vi "UHR-Fleezers Control (host) - 10.7.vi"() -> ()   [LabVIEW 2010] (continued)
          }
        }
        "Raster Scanning..." <- TRUE ("Scanning...")
      }
    }
    n290 = And(x="Save scans", y=w1174) -> (x .and. y?=w1220:bool)
    n291 = Compound Arithmetic op=OR("Start MCL Scan", "Confocal Image", "Confocal Linescan") -> (w1172:bool)
    n292 = And(x="Save Data (MCL)", y=w1172) -> (x .and. y?=w1219:bool)
    n293 = case "Start MCL raster scan" shown="True" w1172 {
      tunnel: w1222 -> [w2230 w2245]
      tunnel: w1221 -> [w2229 w2244]
      tunnel: [w2230 w2240] -> w979
      tunnel: [w2229 w2239] -> w978
      tunnel: [FALSE w2238] -> w1205
      tunnel: "Start MCL Scan" -> [_ w2233]
      tunnel: "Confocal Image" -> [_ w2232]
      tunnel: "Confocal Linescan" -> [_ _]
      frame False {
      }
      frame True {
        w2238 = TRUE
        n294 = case shown="True" "Restart DMA? (MCL)" {
          tunnel: [w2490 w2492] -> w2243
          tunnel: [w2489 w2491] -> w2242
          tunnel: w2245 -> [w2490 w2495]
          tunnel: w2244 -> [w2489 w2494]
          frame False {
          }
          frame True {
            n295 = call "reset FPGA DMA.vi"("error in"=w2494, "FPGA VI Reference In"=w2495) -> ("error out"=w2491:errorcluster, "FPGA VI Reference Out"=w2492:T19)
            n296 = local write "Overflow (data lost)"(FALSE ("Overflow (data lost)")) -> ()
          }
        }
        n297 = case shown="False" w2233 {
          selector: w2233 -> [_ w2249]
          tunnel: w2232 -> [w2248 _]
          tunnel: [w2248 w2249] -> w2231
          frame False {
            n298 = property on="2D or 1D Scan" class="Bool (strict)"("Val(Sgnl)"=w2248) -> ()  [unwired: 2 in, 2 out]
            n299 = property on="Confocal Image" class="Bool (strict)"("Value"=FALSE ("Start Confocal Map")) -> ()  [unwired: 2 in, 2 out]
          }
          frame True {
          }
        }
        n300 = local write "MCL Scanning"(w2238) -> ()
        n301 = local read "AO1"() -> (w2235:dbl)
        n302 = local read "AO2"() -> (w2234:dbl)
        n303 = case shown="True" "Center Scan" {
          tunnel: w2243 -> [w2256 w2368]
          tunnel: w2242 -> [w2255 w2367]
          tunnel: [w2254 w2366] -> w2240
          tunnel: [w2253 w2365] -> w2239
          tunnel: [w2251 w2352] -> w2237
          tunnel: [w2250 w2351] -> w2236
          tunnel: w2235 -> [w2251 w2357]
          tunnel: w2234 -> [w2250 w2360]
          tunnel: w2231 -> [_ _]
          frame False {
            w2252 = TRUE ("AI to FIFO")
            n304 = xnode "Read/Write Control"("FPGA VI Reference In"=w2256, "error in"=w2255, "AI to FIFO"=w2252, "APD to FIFO"=w2252, "Start scan (MCL)"=w2252) -> ("FPGA VI Reference Out"=w2254:T19, "error out"=w2253:errorcluster)
          }
          frame True {
            w2364 = TRUE ("AI to FIFO")
            n305 = local read "Scan steps (MCL)"() -> (w2343:u64)
            n306 = local read "Scan lines (y)"() -> (w2339:u64)
            n307 = local read "Fast Scan Dir"() -> (w2350:bool)
            n308 = local read "Actual MCL Inc (V)"() -> (w2340:dbl)
            n309 = Decrement(x=w2339) -> (x-1=w2338:u64)
            n310 = Decrement(x=w2343) -> (x-1=w2342:u64)
            n311 = Multiply(x=w2340, y=w2338) -> (x*y=w2337:dbl)
            n312 = Divide(x=w2337, y=2.0) -> (x/y=w2347:dbl)
            n313 = Multiply(x=w2340, y=w2342) -> (x*y=w2341:dbl)
            n314 = Divide(x=w2341, y=2.0) -> (x/y=w2346:dbl)
            n315 = Select(t=w2346, s=w2350, f=w2347) -> (s? t:f=w2345:dbl)
            n316 = Select(t=w2347, s=w2350, f=w2346) -> (s? t:f=w2349:dbl)
            n317 = Subtract(x=w2357, y=w2349) -> (x-y=w2348:dbl)
            n318 = Subtract(x=w2360, y=w2345) -> (x-y=w2344:dbl)
            n319 = local read "2D or 1D Scan"() -> (w2362:bool)
            n320 = Not(x=w2350) -> (.not. x?=w2356:bool)
            n321 = Not(x=w2362) -> (.not. x?=w2358:bool)
            n322 = And(x=w2350, y=w2358) -> (x .and. y?=w2359:bool)
            n323 = And(x=w2358, y=w2356) -> (x .and. y?=w2361:bool)
            n324 = Select(t=w2360, s=w2361, f=w2344) -> (s? t:f=w2351:dbl)
            n325 = Select(t=w2357, s=w2359, f=w2348) -> (s? t:f=w2352:dbl)
            n326 = call "Volt to I16.vi"("Voltage In"=w2352) -> ("I16 Voltage Out"=w2355:i16)
            n327 = call "Volt to I16.vi"("Voltage In"=w2351) -> ("I16 Voltage Out"=w2354:i16)
            n328 = xnode "Read/Write Control"("FPGA VI Reference In"=w2368, "error in"=w2367, "AI to FIFO"=w2364, "APD to FIFO"=w2364, "Start scan (MCL)"=w2364, "AO1"=w2355, "AO2"=w2354) -> ("FPGA VI Reference Out"=w2366:T19, "error out"=w2365:errorcluster)
          }
        }
        "Initial Y" <- w2237
        "Initial X" <- w2236
        "wait to reset values" <- w2238
      }
    }
    n329 = local read "Trap Pos Elements/DMA read"() -> (w1053:u32)
    n330 = local read "Trap AI Elements/DMA read"() -> (w977:u32)
    n331 = local read "APD Elements/DMA read"() -> (w1096:u32)
    n332 = local read "Trap AI FIFO Depth"() -> (w1269:u32)
    n333 = xnode "Invoke Method"("FPGA VI Reference In"=w979, "error in"=w978, "Number of Elements"=w1053, "Timeout (ms)"=-1) -> ("Data"=w1017:u16[], "Elements Remaining"=→"Trap Pos FIFO El Remaining":u32)  [unwired: 2 out]
    n334 = xnode "Invoke Method"("FPGA VI Reference In"=w979, "error in"=w978, "Number of Elements"=w977, "Timeout (ms)"=-1 ("Timeout")) -> ("FPGA VI Reference Out"=w981:T19, "error out"=w980:errorcluster, "Data"=w976:i16[], "Elements Remaining"=w982:u32)
    "Trap AI FIFO El. Rem." <- w982
    n335 = xnode "Get APD Data"("FPGA VI Reference In"=w979, "error in"=w978, "Number of Elements"=w1096, "Timeout (ms)"=-1) -> ("Data"=w1095:u32[], "Elements Remaining"=→"APD FIFO Elements Remaining":u32)  [unwired: 2 out]
    n336 = Subtract(x=w1269, y=w977) -> (x-y=w1268:u32)
    n337 = Decimate 1D Array(w1017) -> (w1014:u16[], w1016:u16[], w1015:u16[])
    n338 = Divide(x=w982, y=w1268) -> (x/y=w1267:dbl)
    "Buffer Status" <- w1267
    n339 = To Unsigned Long Integer(number=w1014) -> (unsigned 32bit integer=w1013:u32[])
    n340 = Join Numbers(hi=w1016, lo=w1015) -> ((hi.lo)=w1012:u32[])
    n341 = Equal?(x=w1267, y=1.0) -> (x = y?=w1265:bool)
    n342 = Join Numbers(hi=w1013, lo=w1012) -> ((hi.lo)=w1006:u64[])
    n343 = call "IR AOM word to freq - vec.vi"("Frequency Word In (double vec)"=w1006) -> ("Frequency Out"=w1052:dbl[])
    n344 = case "Alert buffer overflow" shown="True" w1265 {
      frame False {
      }
      frame True {
        n345 = call <vilib>:"Beep.vi"() -> ()  [unwired: 3 in, 9 out]
        "Overflow (data lost)" <- TRUE ("Overflow (data lost)")
      }
    }
    n346 = Decimate 1D Array(w1052) -> (w1051:dbl[], w1050:dbl[])
    n347 = Array Size(array=w976) -> (size(s)=→"Waveform Chart":i32)
    n348 = Build Array(w1051, w1050) -> (w1049:dbl[][])
    n349 = local read "Trap Sets"() -> (w1133:u32)
    n350 = case "Deinterlace trap data, average down PSD" shown="2" w1133 {
      tunnel: w976 -> [w2525 w2590]
      tunnel: [w2522 w2587] -> w1126
      tunnel: [w2525 w2589] -> w1009
      tunnel: "Detector Type" -> [w2524 w2585]
      tunnel: [w2523 w2588] -> w1125
      tunnel: [w2521 w2586] -> w1240
      frame 1, Default {
        n351 = Divide(x=w2525, y=3276.7) -> (x/y=w2526:dbl[])
        n352 = Decimate 1D Array(w2526) -> (w2535:dbl[], w2534:dbl[], w2533:dbl[], w2532:dbl[], w2531:dbl[], w2530:dbl[], w2529:dbl[], w2528:dbl[])
        n353 = case shown="\"IR-QPD + PSD + FB-QPD position\"" w2524 {
          tunnel: w2535 -> [w2559 w2584]
          tunnel: w2534 -> [w2558 w2583]
          tunnel: w2533 -> [w2543 w2561]
          tunnel: w2532 -> [w2544 w2571]
          tunnel: w2531 -> [w2557 w2582]
          tunnel: w2530 -> [w2556 w2581]
          tunnel: w2529 -> [w2540 w2562]
          tunnel: w2528 -> [w2539 w2560]
          tunnel: [w2538 w2568] -> w2523
          tunnel: [w2537 w2567] -> w2522
          tunnel: [w2536 w2566] -> w2521
          frame "IR-QPD + PSD + FB-QPD", Default {
            w2536 = 0  # Channel pattern
            n354 = Divide(x=w2559, y=w2544) -> (x/y=w2546:dbl[])
            n355 = Divide(x=w2558, y=w2544) -> (x/y=w2545:dbl[])
            n356 = Divide(x=w2557, y=w2540) -> (x/y=w2542:dbl[])
            n357 = Divide(x=w2556, y=w2539) -> (x/y=w2541:dbl[])
            n358 = Build Array(w2546, w2545, w2544, w2543, w2542, w2541, w2540, w2539) -> (w2537:dbl[][])
            n359 = Bundle("T1 Y", "T1 X", "T1 Sum", "FB Sum", "PSD Y", "PSD X", "PSD Y Sum", "PSD X Sum") -> (w2555:T40)  [unwired: 1 out]
            n360 = Cluster To Array(cluster=w2555) -> (array=w2538:string[])
          }
          frame "IR-QPD + PSD + FB-QPD position" {
            w2566 = 3  # Channel pattern
            n361 = Negate(x=w2562) -> (-x=w2563:dbl[])
            n362 = Divide(x=w2584, y=w2571) -> (x/y=w2573:dbl[])
            n363 = Divide(x=w2583, y=w2571) -> (x/y=w2572:dbl[])
            n364 = Divide(x=w2582, y=w2562) -> (x/y=w2570:dbl[])
            n365 = Divide(x=w2581, y=w2563) -> (x/y=w2569:dbl[])
            n366 = Build Array(w2573, w2572, w2571, w2560, w2561, w2570, w2569, w2562) -> (w2567:dbl[][])
            n367 = Bundle("T1 Y", "T1 X", "T1 Sum", "FB X", "FB Sum", "PSD Y", "PSD X", "PSD Y Sum") -> (w2580:T40)  [unwired: 1 out]
            n368 = Cluster To Array(cluster=w2580) -> (array=w2568:string[])
          }
        }
      }
      frame 2 {
        n369 = case shown="\"UCB Fleezers 052511\"" w2585 {
          tunnel: w2590 -> [w2652 w2719 w2747 w2854]
          tunnel: [w2591 w2711 w2742 w2785] -> w2589
          tunnel: [w2618 w2702 w2744 w2832] -> w2588
          tunnel: [w2617 w2666 w2721 w2799] -> w2587
          tunnel: [w2611 w2701 w2784 w2830] -> w2586
          frame "IR-QPD + PSD + FB-QPD", Default {
            w2611 = 1  # Channel pattern
            # "time average x2 the 4th signal and the 4 psd signals (detection laser)"
            # "deinterlace 3 signals from qpd"
            n370 = Decimate 1D Array(w2652) -> (w2651:i16[], w2650:i16[], w2616:i16[], w2649:i16[], w2639:i16[], w2637:i16[], w2636:i16[], w2634:i16[])
            n371 = call "downsample 1D array - double.vi"("Ave N"=2.0, "Array In"=w2639) -> ("Array Out"=w2638:dbl[])  [unwired: 1 out]
            n372 = call "downsample 1D array - double.vi"("Ave N"=2.0, "Array In"=w2634) -> ("Array Out"=w2633:dbl[])  [unwired: 1 out]
            n373 = call "downsample 1D array - double.vi"("Ave N"=2.0, "Array In"=w2636) -> ("Array Out"=w2635:dbl[])  [unwired: 1 out]
            n374 = call "downsample 1D array - double.vi"("Ave N"=2.0, "Array In"=w2637) -> ("Array Out"=w2619:dbl[])  [unwired: 1 out]
            n375 = Decimate 1D Array(w2651) -> (w2648:i16[], w2620:i16[])
            n376 = Decimate 1D Array(w2650) -> (w2647:i16[], w2645:i16[])
            n377 = Decimate 1D Array(w2649) -> (w2646:i16[], w2644:i16[])
            n378 = Decimate 1D Array(w2616) -> (w2615:i16[], w2614:i16[])
            n379 = Interleave 1D Arrays(w2648, w2647, w2646, w2620, w2645, w2644, w2615, w2614, w2638, w2619, w2635, w2633) -> (w2632:dbl[])
            n380 = To Word Integer(number=w2632) -> (16bit integer=w2591:i16[])
            n381 = Divide(x=w2632, y=3276.7) -> (x/y=w2631:dbl[])
            n382 = Decimate 1D Array(w2631) -> (w2630:dbl[], w2629:dbl[], w2628:dbl[], w2627:dbl[], w2626:dbl[], w2625:dbl[], w2613:dbl[], w2612:dbl[], w2624:dbl[], w2623:dbl[], w2622:dbl[], w2621:dbl[])
            n383 = Divide(x=w2630, y=w2628) -> (x/y=w2598:dbl[])
            n384 = Divide(x=w2629, y=w2628) -> (x/y=w2597:dbl[])
            n385 = Divide(x=w2627, y=w2625) -> (x/y=w2596:dbl[])
            n386 = Divide(x=w2626, y=w2625) -> (x/y=w2595:dbl[])
            n387 = Divide(x=w2624, y=w2622) -> (x/y=w2594:dbl[])
            n388 = Divide(x=w2623, y=w2621) -> (x/y=w2593:dbl[])
            n389 = Bundle("T1 Y", "T1 X", "T1 Sum", "T2 Y", "T2 X", "T2 Sum", "T1 FB Sum", "T2 FB Sum", "PSD Y", "PSD X", "PSD Y Sum", "PSD X Sum") -> (w2599:T41)  [unwired: 1 out]
            n390 = Build Array(w2598, w2597, w2628, w2596, w2595, w2625, w2613, w2612, w2594, w2593, w2622, w2621) -> (w2617:dbl[][])
            n391 = Cluster To Array(cluster=w2599) -> (array=w2618:string[])
          }
          frame "IR-QPD + PSD + FB-QPD X position" {
            w2701 = 2  # Channel pattern
            # "convert\nADC numbers\nto volts"
            # "time average x2 the 3 psd signals (detection laser)"
            # "deinterlace 3 signals from qpds"
            n392 = Decimate 1D Array(w2719) -> (w2718:i16[], w2717:i16[], w2654:i16[], w2655:i16[], w2664:i16[], w2661:i16[], w2658:i16[], w2689:i16[])
            n393 = Decimate 1D Array(w2718) -> (w2716:i16[], w2703:i16[])
            n394 = call "downsample 1D array - I16.vi"("Ave N"=2.0, "Array In"=w2664) -> ("Array Out"=w2662:i16[])  [unwired: 1 in]
            n395 = call "downsample 1D array - I16.vi"("Ave N"=2.0, "Array In"=w2661) -> ("Array Out"=w2659:i16[])  [unwired: 1 in]
            n396 = Decimate 1D Array(w2717) -> (w2715:i16[], w2713:i16[])
            n397 = Decimate 1D Array(w2655) -> (w2714:i16[], w2712:i16[])
            n398 = Decimate 1D Array(w2689) -> (w2688:i16[], w2686:i16[])
            n399 = Decimate 1D Array(w2654) -> (w2687:i16[], w2685:i16[])
            n400 = call "downsample 1D array - I16.vi"("Ave N"=2.0, "Array In"=w2658) -> ("Array Out"=w2656:i16[])  [unwired: 1 in]
            n401 = Interleave 1D Arrays(w2716, w2715, w2714, w2703, w2713, w2712, w2688, w2687, w2686, w2685, w2662, w2659, w2656) -> (w2711:i16[])
            n402 = Divide(x=w2711, y=3276.7) -> (x/y=w2710:dbl[])
            n403 = Decimate 1D Array(w2710) -> (w2709:dbl[], w2708:dbl[], w2707:dbl[], w2706:dbl[], w2705:dbl[], w2704:dbl[], w2677:dbl[], w2675:dbl[], w2674:dbl[], w2672:dbl[], w2671:dbl[], w2670:dbl[], w2667:dbl[])
            n404 = Divide(x=w2709, y=w2707) -> (x/y=w2693:dbl[])
            n405 = Divide(x=w2708, y=w2707) -> (x/y=w2692:dbl[])
            n406 = Divide(x=w2706, y=w2704) -> (x/y=w2691:dbl[])
            n407 = Divide(x=w2705, y=w2704) -> (x/y=w2690:dbl[])
            n408 = Divide(x=w2677, y=w2675) -> (x/y=w2676:dbl[])
            n409 = Divide(x=w2674, y=w2672) -> (x/y=w2673:dbl[])
            n410 = Divide(x=w2671, y=w2667) -> (x/y=w2669:dbl[])
            n411 = Negate(x=w2667) -> (-x=w2665:dbl[])
            n412 = Divide(x=w2670, y=w2665) -> (x/y=w2668:dbl[])
            n413 = Bundle("T1 Y", "T1 X", "T1 Sum", "T2 Y", "T2 X", "T2 Sum", "T1 FB X", "T1 FB Sum", "T2 FB X", "T2 FB Sum", "PSD Y", "PSD X", "PSD Y Sum") -> (w2694:T42)  [unwired: 1 out]
            n414 = Build Array(w2693, w2692, w2707, w2691, w2690, w2704, w2676, w2675, w2673, w2672, w2669, w2668, w2667) -> (w2666:dbl[][])
            n415 = Cluster To Array(cluster=w2694) -> (array=w2702:string[])
          }
          frame "UCB Fleezers 052511" {
            w2784 = 2  # Channel pattern
            n416 = Decimate 1D Array(w2747) -> (w2782:i16[], w2781:i16[], w2746:i16[], w2745:i16[], w2739:i16[], w2736:i16[], w2735:i16[], w2734:i16[])
            n417 = Decimate 1D Array(w2782) -> (w2780:i16[], w2765:i16[])
            n418 = Decimate 1D Array(w2781) -> (w2779:i16[], w2777:i16[])
            n419 = Decimate 1D Array(w2746) -> (w2778:i16[], w2776:i16[])
            n420 = Decimate 1D Array(w2745) -> (w2741:i16[], w2740:i16[])
            n421 = Decimate 1D Array(w2739) -> (w2738:i16[], w2737:i16[])
            n422 = call "downsample 1D array - I16.vi"("Ave N"=2.0, "Array In"=w2736) -> ("Array Out"=w2733:i16[])  [unwired: 1 in]
            n423 = call "downsample 1D array - I16.vi"("Ave N"=2.0, "Array In"=w2735) -> ("Array Out"=w2732:i16[])  [unwired: 1 in]
            n424 = call "downsample 1D array - I16.vi"("Ave N"=2.0, "Array In"=w2734) -> ("Array Out"=w2731:i16[])  [unwired: 1 in]
            n425 = Interleave 1D Arrays(w2780, w2779, w2778, w2765, w2777, w2776, w2741, w2738, w2740, w2737, w2733, w2732, w2731) -> (w2742:i16[])
            n426 = Divide(x=w2742, y=3276.7) -> (x/y=w2772:dbl[])
            n427 = Decimate 1D Array(w2772) -> (w2771:dbl[], w2770:dbl[], w2769:dbl[], w2768:dbl[], w2767:dbl[], w2766:dbl[], w2730:dbl[], w2728:dbl[], w2727:dbl[], w2725:dbl[], w2724:dbl[], w2723:dbl[], w2722:dbl[])
            n428 = Divide(x=w2771, y=w2769) -> (x/y=w2752:dbl[])
            n429 = Divide(x=w2770, y=w2769) -> (x/y=w2751:dbl[])
            n430 = Divide(x=w2768, y=w2766) -> (x/y=w2750:dbl[])
            n431 = Divide(x=w2767, y=w2766) -> (x/y=w2749:dbl[])
            n432 = Divide(x=w2730, y=w2728) -> (x/y=w2729:dbl[])
            n433 = Divide(x=w2727, y=w2725) -> (x/y=w2726:dbl[])
            n434 = Bundle("T1 Y", "T1 X", "T1 Sum", "T2 Y", "T2 X", "T2 Sum", "T1 FB X", "T2 FB Sum", "T2 FB X", "T2 FB Sum", "PSD Y", "PSD X", "PSD Sum") -> (w2753:T42)  [unwired: 1 out]
            n435 = Build Array(w2752, w2751, w2769, w2750, w2749, w2766, w2729, w2728, w2726, w2725, w2724, w2723, w2722) -> (w2721:dbl[][])
            n436 = Cluster To Array(cluster=w2753) -> (array=w2744:string[])
          }
          frame "IR-QPD + PSD + FB-QPD XY positions" {
            w2830 = 4  # Channel pattern
            # "time average x2 the 3 psd signals (detection laser)"
            # "deinterlace 3 signals from qpds"
            n437 = Decimate 1D Array(w2854) -> (w2853:i16[], w2852:i16[], w2831:i16[], w2851:i16[], w2797:i16[], w2843:i16[], w2842:i16[], w2819:i16[])
            n438 = Decimate 1D Array "QPD Y"(w2853) -> (w2850:i16[], w2833:i16[])
            n439 = call "downsample 1D array - double.vi"("Ave N"=2.0, "Array In"=w2843) -> ("Array Out"=w2818:dbl[])  [unwired: 1 out]
            n440 = call "downsample 1D array - double.vi"("Ave N"=2.0, "Array In"=w2842) -> ("Array Out"=w2817:dbl[])  [unwired: 1 out]
            n441 = Decimate 1D Array "Feedback Sum"(w2831) -> (w2815:i16[], w2813:i16[])
            n442 = Decimate 1D Array "Feedback Y"(w2797) -> (w2796:i16[], w2795:i16[])
            n443 = Decimate 1D Array "Feedback X"(w2819) -> (w2816:i16[], w2814:i16[])
            n444 = Decimate 1D Array "QPD Sum"(w2851) -> (w2848:i16[], w2846:i16[])
            n445 = Decimate 1D Array "QPD X"(w2852) -> (w2849:i16[], w2847:i16[])
            n446 = Interleave 1D Arrays(w2850, w2849, w2848, w2833, w2847, w2846, w2796, w2816, w2815, w2795, w2814, w2813, w2818, w2817) -> (w2841:dbl[])
            n447 = To Word Integer(number=w2841) -> (16bit integer=w2785:i16[])
            n448 = Divide(x=w2841, y=3276.7) -> (x/y=w2840:dbl[])
            n449 = Decimate 1D Array(w2840) -> (w2839:dbl[], w2838:dbl[], w2837:dbl[], w2836:dbl[], w2835:dbl[], w2834:dbl[], w2792:dbl[], w2806:dbl[], w2790:dbl[], w2791:dbl[], w2804:dbl[], w2788:dbl[], w2802:dbl[], w2800:dbl[])
            n450 = Divide(x=w2839, y=w2837) -> (x/y=w2823:dbl[])
            n451 = Divide(x=w2838, y=w2837) -> (x/y=w2822:dbl[])
            n452 = Divide(x=w2836, y=w2834) -> (x/y=w2821:dbl[])
            n453 = Divide(x=w2835, y=w2834) -> (x/y=w2820:dbl[])
            n454 = Divide(x=w2792, y=w2790) -> (x/y=w2789:dbl[])
            n455 = Divide(x=w2806, y=w2790) -> (x/y=w2805:dbl[])
            n456 = Divide(x=w2791, y=w2788) -> (x/y=w2787:dbl[])
            n457 = Divide(x=w2804, y=w2788) -> (x/y=w2803:dbl[])
            n458 = Negate(x=w2800) -> (-x=w2798:dbl[])
            n459 = Divide(x=w2802, y=w2798) -> (x/y=w2801:dbl[])
            n460 = Bundle("T1 Y", "T1 X", "T1 Sum", "T2 Y", "T2 X", "T2 Sum", "T1 FB Y", "T1 FB X", "T1 FB Sum", "T2 FB Y", "T2 FB X", "T2 FB Sum", "PSD X", "PSD Y Sum") -> (w2786:T43)  [unwired: 1 out]
            n461 = Build Array(w2823, w2822, w2837, w2821, w2820, w2834, w2789, w2805, w2790, w2787, w2803, w2788, w2801, w2800) -> (w2799:dbl[][])
            n462 = Cluster To Array(cluster=w2786) -> (array=w2832:string[])
          }
        }
      }
    }
    "AI labels" <- w1125
    n463 = Decimate 1D Array(w1095) -> (w1123:u32[], w1059:u32[])
    n464 = local read "DMA Update Period (s)"() -> (w1134:dbl)
    n465 = local read "BD 1 Frequency 2 (MHz)"() -> (w1001:dbl)
    n466 = local read "BD 1 Frequency 1 (MHz)"() -> (w1002:dbl)
    n467 = Build Array(w1123, w1059) -> (w1202:u32[][])
    n468 = local read "Data Period (s)"() -> (w1108:dbl)
    n469 = Decimate 1D Array(w1009) -> (w1032:i16[], w1031:i16[], w1029:i16[], w1028:i16[])  [unwired: 9 out]
    n470 = To Double Precision Float(number=w1202) -> (double precision float=w1203:dbl[][])
    n471 = local read "APD Integration Time (s)"() -> (w1072:dbl)
    n472 = Divide(x=w1032, y=w1031) -> (x/y=w1033:dbl[])
    n473 = Divide(x=w1029, y=w1028) -> (x/y=w1030:dbl[])
    n474 = feedback #1(0.0) -> (w1046:dbl)
    n475 = Add(x=w1134, y=w1046) -> (x+y=w1242:dbl)
    n476 = feedback-in #1(w1242) -> ()
    n477 = local read "AOM X Cal (nm/MHz)"() -> (w999:dbl)
    n478 = To Time Stamp(1:w1046) -> (0:w1045:timestamp)
    n479 = Split 1D Array(array=w1033, index="N El. to Ave.") -> (second subarray=w1036:dbl[])  [unwired: 1 out]
    n480 = Split 1D Array(array=w1030, index="N El. to Ave.") -> (second subarray=w1035:dbl[])  [unwired: 1 out]
    n481 = local read "Trap X AI1 (DMA)"() -> (w1034:T13)
    n482 = Multiply(x=w1108, y="Trap Disp. Downsample") -> (x*y=w1047:dbl)
    "Display Period (s)" <- w1047
    n483 = Bundle("BD 1 Frequency 1 (MHz)"=w1002, "BD 1 Frequency 2 (MHz)"=w1001) -> (w1003:T44)  [unwired: 1 out]
    n484 = for "Trap AI" {
      tunnel: [w2520] -> w1236 mode=indexing
      tunnel: w1045 -> [w2510]
      tunnel: "Trap Disp. Downsample" -> [w2518]
      tunnel: w1126 -> [w2516] mode=indexing
      tunnel: w1108 -> [w2515]
      tunnel: w1125 -> [w2514] mode=indexing
      tunnel: w1044 -> [w2513]
      tunnel: [w2512] -> w1083 mode=indexing
      tunnel: w1047 -> [w2511]
      n485 = Bundle By Name("Y"=w2516, "dt"=w2515) -> (w2517:waveform(dbl))  [unwired: 1 out]
      n486 = Set Waveform Attribute(5:w2514, 6:w2513, 7:w2517) -> (3:w2512:waveform(dbl))  [unwired: 1 in, 2 out]
      n487 = call "downsample 1D array - double.vi"("Ave N"=w2518, "Array In"=w2516) -> ("Array Out"=w2519:dbl[])  [unwired: 1 out]
      n488 = Bundle By Name(cluster=w2512, "t0"=w2510, "Y"=w2519, "dt"=w2511) -> (w2520:waveform(dbl))
    }
    n489 = call <vilib>:"Mean.vi"("X"=w1035) -> ("mean"=w1023:dbl)  [unwired: 1 out]
    n490 = call <vilib>:"Mean.vi"("X"=w1036) -> ("mean"=w1024:dbl)  [unwired: 1 out]
    n491 = Cluster To Array(cluster=w1003) -> (array=w1000:dbl[])
    n492 = Reciprocal(x=w1047) -> (1/x=→"Trap Disp. Freq. (Hz)":dbl)
    n493 = local read "Data points/scans (MCL)"() -> (w1214:dbl)
    n494 = To Fixed-Point(number=w1023) -> (fixed-point=w1021:fxp<+/-,16,1>)  [unwired: 1 in]
    n495 = To Fixed-Point(number=w1024) -> (fixed-point=w1022:fxp<+/-,16,1>)  [unwired: 1 in]
    n496 = Bundle("Trap 1 Pos.", "Trap 2 Pos.") -> (w1043:cluster{string, string})  [unwired: 1 out]
    n497 = Bundle By Name(cluster=w1034, "Set 1"=w1022, "Set 2"=w1021) -> (→"Trap X AI1 (DMA)":T13)
    n498 = Cluster To Array(cluster=w1043) -> (array=w1040:string[])
    n499 = for "Trap Position" {
      tunnel: w1049 -> [w1497] mode=indexing
      tunnel: "Trap Disp. Downsample" -> [w1496]
      tunnel: w1047 -> [w1494]
      tunnel: w1045 -> [w1493]
      tunnel: w1044 -> [w1491]
      tunnel: w1040 -> [w1490] mode=indexing
      tunnel: [w1489] -> w998 mode=indexing
      tunnel: w1000 -> [w1487] mode=indexing
      tunnel: w999 -> [w1485]
      n500 = call "downsample 1D array - double.vi"("Ave N"=w1496, "Array In"=w1497) -> ("Array Out"=w1495:dbl[])  [unwired: 1 out]
      n501 = Subtract(x=w1495, y=w1487) -> (x-y=w1488:dbl[])
      n502 = Multiply(x=w1485, y=w1488) -> (x*y=w1486:dbl[])
      n503 = Bundle By Name("Y"=w1486, "dt"=w1494, "t0"=w1493) -> (w1492:waveform(dbl))  [unwired: 1 out]
      n504 = Set Waveform Attribute(5:w1490, 6:w1491, 7:w1492) -> (3:w1489:waveform(dbl))  [unwired: 1 in, 2 out]
    }
    "Trap Positions" <- w998
    n505 = Bundle("APD 1", "APD 2") -> (w1235:cluster{string, string})  [unwired: 1 out]
    n506 = Cluster To Array(cluster=w1235) -> (array=w1232:string[])
    n507 = for "APD" {
      tunnel: w1203 -> [w2499] mode=indexing
      tunnel: w1072 -> [w2507]
      tunnel: [w2503] -> w1079 mode=indexing
      tunnel: "APD Disp. Scale" -> [w2504]
      tunnel: w1044 -> [w2502]
      tunnel: w1232 -> [w2501] mode=indexing
      tunnel: "APD Disp. Downsample" -> [w2497]
      tunnel: [w2500] -> w1231
      tunnel: w1045 -> [w2496]
      n508 = call "integrate 1D array interval - double.vi"("Ave N"=w2497, "Array In"=w2499) -> ("Array Out"=w2498:dbl[])  [unwired: 1 out]
      n509 = Multiply(x=w2507, y=w2497) -> (x*y=w2500:dbl)
      n510 = Divide(x=w2498, y=w2504) -> (x/y=w2505:dbl[])
      n511 = Bundle By Name("t0"=w2496, "Y"=w2505, "dt"=w2500) -> (w2506:waveform(dbl))  [unwired: 1 out]
      n512 = Set Waveform Attribute(5:w2501, 6:w2502, 7:w2506) -> (3:w2503:waveform(dbl))  [unwired: 1 in, 2 out]
    }
    "APD Display Period (s)" <- w1231
    n513 = Reciprocal(x=w1231) -> (1/x=→"APD Display Freq. (Hz)":dbl)
    n514 = local read "Display Period (s)"() -> (w1107:dbl)
    n515 = Increment(x=w1214) -> (x+1=w1215:dbl)
    n516 = Index Array(array=w998, index=0) -> (element=w996:waveform(dbl))
    n517 = To Double Precision Float(number=w1123) -> (double precision float=w1122:dbl[])
    n518 = feedback #2(w1215) -> (w1218:dbl)
    n519 = Select(t=0, s=w1205, f=w1218) -> (s? t:f=w1211:dbl)
    n520 = Array Size(array=w1122) -> (size(s)=w1217:i32)
    n521 = Add(x=w1217, y=w1211) -> (x+y=w1212:dbl)
    n522 = Unbundle By Name(w996) -> ("Y"=w994:dbl[])
    n523 = feedback #3(w1123) -> (w1201:u32[])
    n524 = Build Array (concatenate)(w1201, w1123) -> (w1198:u32[])
    n525 = feedback #4(w1059) -> (w1078:u32[])
    n526 = Divide(x="Bead Sep. Int. Time (s)", y=w1107) -> (x/y=w992:dbl)
    n527 = Build Array (concatenate)(w1078, w1059) -> (w1077:u32[])
    n528 = Greater?(x=w1212, y=w1214) -> (0:w1213:bool)
    n529 = feedback #5(w994) -> (w995:dbl[])
    n530 = Build Array (concatenate)(w994, w995) -> (w993:dbl[])
    n531 = Select(t=w1211, s=w1213, f=w1212) -> (s? t:f=w1210:dbl)
    n532 = feedback-in #2(w1210) -> ()
    n533 = Array Size(array=w1198) -> (size(s)=w1195:i32)
    n534 = Array Size(array=w1123) -> (size(s)=w1197:i32)
    n535 = local read "MCL Scanning"() -> (w1208:bool)
    n536 = local read "APD Integration Time (s)"() -> (w1086:dbl)
    n537 = Build Array (concatenate)(w1079, w1236) -> (w1081:waveform(dbl)[])
    "All Signals" <- w1081
    n538 = Split 1D Array(array=w993, index=w992) -> (first subarray=w986:dbl[])  [unwired: 1 out]
    n539 = feedback-in #5(w986) -> ()
    n540 = Multiply(x=w1197, y="APD Ave N") -> (x*y=w1196:dbl)
    n541 = Greater?(x=w1195, y=w1196) -> (0:w1199:bool)
    n542 = Not(x=w1213) -> (.not. x?=w1207:bool)
    n543 = To Double Precision Float(number=w1059) -> (double precision float=w1058:dbl[])
    n544 = call <vilib>:"Mean.vi"("X"=w986) -> ("mean"=w985:dbl)  [unwired: 1 out]
    "Mean T1 Position (nm)" <- w985
    n545 = Subtract(x=w986, y=w985) -> (x-y=w991:dbl[])
    n546 = Square(x=w991) -> (x^2=w990:dbl[])
    n547 = And(x=w1207, y=w1208) -> (x .and. y?=w1209:bool)
    n548 = call <vilib>:"Mean.vi"("X"=w990) -> ("mean"=w989:dbl)  [unwired: 1 out]
    n549 = case shown="True" w1199 {
      tunnel: w1198 -> [w2080 w2087]
      tunnel: [w2080 w2085] -> w1139
      tunnel: w1196 -> [_ w2082]
      tunnel: w1195 -> [_ w2086]
      tunnel: w1077 -> [w2079 w2084]
      tunnel: [w2079 w2081] -> w1074
      frame False {
      }
      frame True {
        n550 = Subtract(x=w2086, y=w2082) -> (x-y=w2083:dbl)
        n551 = Array Subset(array=w2087, index=w2083, length=w2082) -> (w2085:u32[])
        n552 = Array Subset(array=w2084, index=w2083, length=w2082) -> (w2081:u32[])
      }
    }
    n553 = feedback-in #3(w1139) -> ()
    n554 = feedback-in #4(w1074) -> ()
    n555 = Or(x=w1209, y=w1205) -> (x .or. y?=w1206:bool)
    n556 = Square Root(x=w989) -> (sqrt(x)=w988:dbl)
    n557 = Equal?(x="Tab Control 6", y=T32."High Res Display") -> (x = y?=w1129:bool)
    n558 = Multiply(x="APD Disp. Scale", y=w1079) -> (x*y=w1088:waveform(dbl)[])
    n559 = Multiply(x="APD Disp. Downsample", y=w1086) -> (x*y=w1084:dbl)
    n560 = Multiply(x=10.0, y=w988) -> (x*y=→"Trap 1 Position RMS (A)":dbl)
    n561 = Divide(x=w1088, y=w1084) -> (x/y=w1056:waveform(dbl)[])
    n562 = Index Array(array=w1056, index=0) -> (element=w1066:waveform(dbl))
    n563 = case "For computing FFTs for display" shown="True" "Compute FFT" {
      tunnel: w1083 -> [_ w3407]
      frame False {
      }
      frame True {
        n564 = Build Array("FFT 1 Choice 1", "FFT 1 Choice 2", "FFT 2 Choice 1", "FFT 2 Choice 2") -> (w3400:u16[])
        n565 = Array Size(array=w3407) -> (size(s)=w3406:i32)
        n566 = feedback-in #6(w3400) -> ()
        n567 = feedback #6(u16[] [100, 100, 100, 100]) -> (w3401:u16[])
        n568 = feedback-in #7("# Spectra to Ave.") -> ()
        n569 = feedback #7("# Spectra to Ave.") -> (w3398:dbl)
        n570 = Not Equal?(x="# Spectra to Ave.", y=w3398) -> (x != y?=w3397:bool)
        n571 = Not Equal?(x=w3400, y=w3401) -> (x != y?=w3399:bool)
        n572 = feedback #8(1.0) -> (w3384:dbl)
        n573 = Compound Arithmetic op=OR("Reset FFT", w3399, w3397) -> (w3382:bool)
        n574 = Select(t=1.0, s=w3382, f=w3384) -> (s? t:f=w3386:dbl)
        n575 = Greater?(x=w3386, y="# Spectra to Ave.") -> (0:w3405:bool)
        n576 = Increment(x=w3386) -> (x+1=w3385:dbl)
        n577 = feedback-in #8(w3385) -> ()
        n578 = local read "DMA Update Period (s)"() -> (w3380:dbl)
        n579 = Multiply(x="# Spectra to Ave.", y=w3380) -> (x*y=→"Ave. Time (s)":dbl)
        n580 = Build Array(cluster{"f0":dbl, "df":dbl, "magnitude":dbl[]} {"f0"=0.0, "df"=0.0, "magnitude"=[]} ("PSD")) -> (w3389:cluster{"f0":dbl, "df":dbl, "magnitude":dbl[]}[])
        n581 = Build Array(w3389, w3389, w3389, w3389) -> (w3391:T45)
        n582 = feedback #9(w3391) -> (w3396:T45)
        n583 = for {
          N: 4 -> [_]
          tunnel: w3400 -> [w3429] mode=indexing
          tunnel: w3407 -> [w3430]
          tunnel: w3406 -> [w3432]
          tunnel: w3382 -> [w3425]
          tunnel: w3405 -> [w3424]
          tunnel: "# Spectra to Ave." -> [w3423]
          tunnel: [w3422] -> w3395 mode=indexing
          tunnel: w3396 -> [w3427] mode=indexing
          tunnel: [w3426] -> w3383 mode=indexing
          tunnel: w3386 -> [w3421]
          n584 = Less?(x=w3429, y=w3432) -> (x < y?=w3431:bool)
          n585 = Index Array(array=w3430, index=w3429) -> (element=w3428:waveform(dbl))
          n586 = case shown="True" w3431 {
            tunnel: w3428 -> [_ w3449]
            tunnel: w3427 -> [w3434 w3447]
            tunnel: [w3434 w3435] -> w3426
            tunnel: w3425 -> [_ w3446]
            tunnel: w3424 -> [_ w3439]
            tunnel: w3423 -> [_ w3438]
            tunnel: [cluster{"f0":dbl, "df":dbl, "magnitude":dbl[]} {"f0"=0.0, "df"=0.0, "magnitude"=[]} ("PSD") w3440] -> w3422
            tunnel: w3421 -> [_ w3437]
            frame False {
            }
            frame True {
              n587 = call <vilib>:"Std Deviation and Variance.vi"("X"=w3449) -> ("mean"=w3450:dbl)  [unwired: 1 in, 2 out]
              n588 = Subtract(x=w3449, y=w3450) -> (x-y=w3448:waveform(dbl))
              n589 = xnode "Spectral Measurements"("Signals"=w3448) -> ("PSD"=w3442:cluster{"f0":dbl, "df":dbl, "magnitude":dbl[]})  [unwired: 1 in, 1 out]
              n590 = case shown="False" w3446 {
                tunnel: w3447 -> [w3459 _]
                tunnel: [w3455 w3464] -> w3435
                tunnel: w3442 -> [w3458 w3465]
                tunnel: w3439 -> [w3457 _]
                frame False {
                  n591 = Build Array (concatenate)(w3459, w3458) -> (w3456:cluster{"f0":dbl, "df":dbl, "magnitude":dbl[]}[])
                  n592 = case shown="True" w3457 {
                    tunnel: w3456 -> [w3460 w3463]
                    tunnel: [w3460 w3461] -> w3455
                    frame False {
                    }
                    frame True {
                      n593 = Delete From Array(array=w3463, index=0) -> (array with subset deleted=w3461:cluster{"f0":dbl, "df":dbl, "magnitude":dbl[]}[])  [unwired: 1 in, 1 out]
                    }
                  }
                }
                frame True {
                  n594 = Build Array(w3465) -> (w3464:cluster{"f0":dbl, "df":dbl, "magnitude":dbl[]}[])
                }
              }
              n595 = for {
                tunnel: w3435 -> [w3454] mode=indexing
                tunnel: [w3453] -> w3445 mode=indexing
                workers-P: _ -> [_]
                n596 = Unbundle By Name(w3454) -> ("magnitude"=w3453:dbl[])
              }
              n597 = Transpose 2D Array(2D array=w3445) -> (transposed array=w3444:dbl[][])
              n598 = for {
                tunnel: w3444 -> [w3452] mode=indexing
                tunnel: [w3451] -> w3443 mode=indexing
                workers-P: _ -> [_]
                n599 = Add Array Elements(numeric array=w3452) -> (sum=w3451:dbl)
              }
              n600 = Select(t=w3438, s=w3439, f=w3437) -> (s? t:f=w3436:dbl)
              n601 = Divide(x=w3443, y=w3436) -> (x/y=w3441:dbl[])
              n602 = Bundle By Name(cluster=w3442, "magnitude"=w3441) -> (w3440:cluster{"f0":dbl, "df":dbl, "magnitude":dbl[]})
            }
          }
        }
        n603 = case shown="True" w3382 {
          tunnel: w3383 -> [w3414 w3420]
          tunnel: [w3414 w3415] -> w3381
          frame False {
          }
          frame True {
            n604 = Array Subset(array=w3420, index (row)=0 ("index"), length (row)=4 ("length"), index (col)=0 ("index"), length (col)=1 ("length")) -> (w3415:T45)
          }
        }
        n605 = feedback-in #9(w3381) -> ()
        n606 = Split 1D Array(array=w3395, index=2) -> (first subarray=→"FFT 1":cluster{"f0":dbl, "df":dbl, "magnitude":dbl[]}[], second subarray=→"FFT 2":cluster{"f0":dbl, "df":dbl, "magnitude":dbl[]}[])
      }
    }
    n607 = Index Array(array=w1056, index=1) -> (element=w1064:waveform(dbl))
    n608 = case "For displaying the high resolution display (no downsampling)" shown="True" w1129 {
      tunnel: w1083 -> [_ w1589]
      frame False {
      }
      frame True {
        n609 = Index Array(array=w1589, index="High Res. Display") -> (element=w1590:waveform(dbl))
        n610 = call <vilib>:"Std Deviation and Variance.vi"("X"=w1590) -> ("mean"=w1597:dbl, "standard deviation"=w1602:dbl)  [unwired: 1 in, 1 out]
        "Mean Intensity" <- w1597
        "Sigma" <- w1602
        n611 = Subtract(x=w1590, y=w1597) -> (x-y=w1596:waveform(dbl))
        n612 = Select(t=w1596, s="Subtract mean", f=w1590) -> (s? t:f=→"1 Channel":waveform(dbl))
        n613 = Divide(x=w1602, y=w1597) -> (x/y=→"Sigma/Mean":dbl)
        n614 = feedback #10(1) -> (w1591:i32)
        n615 = Greater Or Equal?(x=w1591, y="Slow mean N ave.") -> (x >= y?=w1604:bool)
        n616 = Increment(x=w1591) -> (x+1=w1606:i32)
        n617 = Select(t=1, s=w1604, f=w1606) -> (s? t:f=w1593:i32)
        n618 = feedback-in #10(w1593) -> ()
        n619 = feedback #11() -> (w1594:waveform(dbl))  [unwired: 1 out]
        n620 = case shown="Default" w1591 {
          tunnel: [w1609 w1612] -> w1595
          tunnel: w1594 -> [w1611 _]
          tunnel: w1590 -> [w1610 w1612]
          frame Default {
            n621 = call-poly <vilib>:"Append Waveforms.vi"("waveform B"=w1610, "waveform A"=w1611) -> ("waveform out"=w1609:waveform(dbl))  [unwired: 1 in, 8 out]
          }
          frame 1 {
          }
        }
        n622 = feedback-in #11(w1595) -> ()
        n623 = case shown="True" w1604 {
          tunnel: w1595 -> [_ w1608]
          frame False {
          }
          frame True {
            n624 = call <vilib>:"Mean.vi"("X"=w1608) -> ("mean"=→"Slow mean":dbl)  [unwired: 1 out]
          }
        }
      }
    }
    n625 = case "For plotting results of scanning MCL" shown="True" w1206 {
      tunnel: w1205 -> [_ w2120]
      tunnel: w1122 -> [_ w2216]
      tunnel: w1214 -> [_ _]
      tunnel: w1083 -> [_ w2190]
      tunnel: w1058 -> [_ w2121]
      tunnel: w1057 -> [_ w2094]
      frame False {
      }
      frame True {
        w2101 = u32 0 items=["Horizontal", "Vertical", "Central", "1st Diagonal", "2nd Diagonal"] ("Type of Symmetry")
        w2129 = u32 0 items=["Horizontal", "Vertical", "Central", "1st Diagonal", "2nd Diagonal"] ("Type of Symmetry")
        w2132 = u32 0 items=["Horizontal", "Vertical", "Central", "1st Diagonal", "2nd Diagonal"] ("Type of Symmetry")
        w2161 = u32 0 items=["Horizontal", "Vertical", "Central", "1st Diagonal", "2nd Diagonal"] ("Type of Symmetry")
        n626 = Index Array(array=w2190, index=10) -> (element=w2196:waveform(dbl))
        n627 = Index Array(array=w2190, index=11) -> (element=w2193:waveform(dbl))
        n628 = local read "Cycles/step (MCL)"() -> (w2146:u64)
        n629 = Index Array(array=w2190, index="Channel") -> (element=w2192:waveform(dbl))
        n630 = Unbundle(w2094) -> ("New Image"=w2093:T2, "New Image"=w2092:T2, "New Image"=w2091:T2, "New Image"=w2090:T2)
        n631 = Unbundle By Name(w2196) -> ("Y"=w2148:dbl[])
        n632 = Unbundle By Name(w2193) -> ("Y"=w2150:dbl[])
        n633 = Unbundle By Name(w2192) -> ("Y"=w2155:dbl[])
        n634 = call "downsample 1D array - double.vi"("Ave N"=w2146, "Array In"=w2148) -> ("Array Out"=w2147:dbl[])  [unwired: 1 out]
        n635 = call "downsample 1D array - double.vi"("Ave N"=w2146, "Array In"=w2150) -> ("Array Out"=w2149:dbl[])  [unwired: 1 out]
        n636 = call "downsample 1D array - double.vi"("Ave N"=w2146, "Array In"=w2155) -> ("Array Out"=w2154:dbl[])  [unwired: 1 out]
        n637 = feedback #12(w2216) -> (w2217:dbl[])
        n638 = Build Array (concatenate)(w2217, w2216) -> (w2198:dbl[])
        n639 = feedback #13(w2121) -> (w2123:dbl[])
        n640 = Build Array (concatenate)(w2123, w2121) -> (w2122:dbl[])
        n641 = local read "Scan steps (MCL)"() -> (w2103:u64)
        n642 = Select(t=w2216, s=w2120, f=w2198) -> (s? t:f=w2202:dbl[])
        n643 = feedback-in #12(w2202) -> ()
        n644 = Select(t=w2121, s=w2120, f=w2122) -> (s? t:f=w2104:dbl[])
        n645 = feedback-in #13(w2104) -> ()
        n646 = local read "Scan lines (y)"() -> (w2089:u64)
        n647 = local read "N APD Samp/step"() -> (w2105:dbl)
        n648 = feedback #14(w2147) -> (w2204:dbl[])
        n649 = Build Array (concatenate)(w2204, w2147) -> (w2195:dbl[])
        n650 = feedback #15(w2154) -> (w2214:dbl[])
        n651 = Build Array (concatenate)(w2214, w2154) -> (w2213:dbl[])
        n652 = feedback #16(w2149) -> (w2206:dbl[])
        n653 = Build Array (concatenate)(w2206, w2149) -> (w2207:dbl[])
        n654 = Select(t=w2147, s=w2120, f=w2195) -> (s? t:f=w2151:dbl[])
        n655 = feedback-in #14(w2151) -> ()
        n656 = Select(t=w2154, s=w2120, f=w2213) -> (s? t:f=w2153:dbl[])
        n657 = feedback-in #15(w2153) -> ()
        n658 = Select(t=w2149, s=w2120, f=w2207) -> (s? t:f=w2152:dbl[])
        n659 = feedback-in #16(w2152) -> ()
        n660 = Multiply(x=w2103, y=u64 2) -> (x*y=w2088:u64)
        n661 = call "integrate 1D array interval - double.vi"("Ave N"=w2105, "Array In"=w2104) -> ("Array Out"=w2116:dbl[])  [unwired: 1 out]
        n662 = call "integrate 1D array interval - double.vi"("Ave N"=w2105, "Array In"=w2202) -> ("Array Out"=w2201:dbl[])  [unwired: 1 out]
        n663 = Array Size(array=w2116) -> (size(s)=w2117:i32)
        n664 = Array Size(array=w2201) -> (size(s)=w2203:i32)
        n665 = Multiply(x=w2089, y=w2088) -> (x*y=w2119:u64)
        n666 = Multiply(x=w2089, y=w2088) -> (x*y=w2211:u64)
        n667 = call <vilib>:"Mean.vi"("X"=w2151) -> ("mean"=w2135:dbl)  [unwired: 1 out]
        n668 = Subtract(x=w2119, y=w2117) -> (x-y=w2110:u64)
        n669 = call <vilib>:"Mean.vi"("X"=w2153) -> ("mean"=w2140:dbl)  [unwired: 1 out]
        n670 = call <vilib>:"Mean.vi"("X"=w2152) -> ("mean"=w2138:dbl)  [unwired: 1 out]
        n671 = call <vilib>:"Mean.vi"("X"=w2116) -> ("mean"=w2107:dbl)  [unwired: 1 out]
        n672 = Subtract(x=w2211, y=w2203) -> (x-y=w2145:u64)
        n673 = call <vilib>:"Mean.vi"("X"=w2201) -> ("mean"=w2142:dbl)  [unwired: 1 out]
        n674 = Initialize Array(1.0 ("element"), w2110) -> (w2106:dbl[])
        n675 = Initialize Array(1.0 ("element"), w2145) -> (w2136:dbl[])
        n676 = Multiply(x=w2106, y=w2107) -> (x*y=w2108:dbl[])
        n677 = Multiply(x=w2136, y=w2138) -> (x*y=w2139:dbl[])
        n678 = Multiply(x=w2136, y=w2140) -> (x*y=w2141:dbl[])
        n679 = Multiply(x=w2136, y=w2135) -> (x*y=w2137:dbl[])
        n680 = Multiply(x=w2136, y=w2142) -> (x*y=w2143:dbl[])
        n681 = Build Array (concatenate)(w2151, w2137) -> (w2205:dbl[])
        n682 = Build Array (concatenate)(w2153, w2141) -> (w2209:dbl[])
        n683 = Build Array (concatenate)(w2152, w2139) -> (w2208:dbl[])
        n684 = Build Array (concatenate)(w2116, w2108) -> (w2118:dbl[])
        n685 = Build Array (concatenate)(w2201, w2143) -> (w2210:dbl[])
        n686 = Reshape Array(w2205, w2089, w2088) -> (w2171:dbl[][])
        n687 = Reshape Array(w2118, w2089, w2088) -> (w2114:dbl[][])
        n688 = Reshape Array(w2209, w2089, w2088) -> (w2163:dbl[][])
        n689 = Reshape Array(w2208, w2089, w2088) -> (w2178:dbl[][])
        n690 = Reshape Array(w2210, w2089, w2088) -> (w2188:dbl[][])
        n691 = Array Subset(array=w2178, index (col)=0 ("index"), length (col)=w2103) -> (w2183:dbl[][])  [unwired: 2 in]
        n692 = Array Subset(array=w2178, index (col)=w2103) -> (w2181:dbl[][])  [unwired: 3 in]
        n693 = Array Subset(array=w2163, index (col)=0 ("index"), length (col)=w2103) -> (w2169:dbl[][])  [unwired: 2 in]
        n694 = Array Subset(array=w2163, index (col)=w2103) -> (w2167:dbl[][])  [unwired: 3 in]
        n695 = Array Subset(array=w2114, index (col)=0 ("index"), length (col)=w2103) -> (w2113:dbl[][])  [unwired: 2 in]
        n696 = Array Subset(array=w2114, index (col)=w2103) -> (w2111:dbl[][])  [unwired: 3 in]
        n697 = Array Subset(array=w2188, index (col)=0 ("index"), length (col)=w2103) -> (w2187:dbl[][])  [unwired: 2 in]
        n698 = Array Subset(array=w2188, index (col)=w2103) -> (w2185:dbl[][])  [unwired: 3 in]
        n699 = Array Subset(array=w2171, index (col)=0 ("index"), length (col)=w2103) -> (w2176:dbl[][])  [unwired: 2 in]
        n700 = Array Subset(array=w2171, index (col)=w2103) -> (w2174:dbl[][])  [unwired: 3 in]
        n701 = for {
          tunnel: w2183 -> [w2225] mode=indexing
          tunnel: [w2224] -> w2182 mode=indexing
          workers-P: _ -> [_]
          n702 = Reverse 1D Array(array=w2225) -> (reversed array=w2224:dbl[])
        }
        n703 = for {
          tunnel: w2169 -> [w2221] mode=indexing
          tunnel: [w2220] -> w2168 mode=indexing
          workers-P: _ -> [_]
          n704 = Reverse 1D Array(array=w2221) -> (reversed array=w2220:dbl[])
        }
        n705 = for {
          tunnel: w2113 -> [w2219] mode=indexing
          tunnel: [w2218] -> w2112 mode=indexing
          workers-P: _ -> [_]
          n706 = Reverse 1D Array(array=w2219) -> (reversed array=w2218:dbl[])
        }
        n707 = for {
          tunnel: w2187 -> [w2227] mode=indexing
          tunnel: [w2226] -> w2186 mode=indexing
          workers-P: _ -> [_]
          n708 = Reverse 1D Array(array=w2227) -> (reversed array=w2226:dbl[])
        }
        n709 = for {
          tunnel: w2176 -> [w2223] mode=indexing
          tunnel: [w2222] -> w2175 mode=indexing
          workers-P: _ -> [_]
          n710 = Reverse 1D Array(array=w2223) -> (reversed array=w2222:dbl[])
        }
        n711 = Index Array(array=w2188, index (row)=0) -> (element=→"Waveform Graph":dbl[])  [unwired: 1 in]
        n712 = Add(x=w2182, y=w2181) -> (x+y=w2180:dbl[][])
        n713 = Add(x=w2168, y=w2167) -> (x+y=w2166:dbl[][])
        n714 = Add(x=w2112, y=w2111) -> (x+y=w2096:dbl[][])
        n715 = Add(x=w2186, y=w2185) -> (x+y=w2160:dbl[][])
        n716 = Add(x=w2175, y=w2174) -> (x+y=w2173:dbl[][])
        n717 = Divide(x=w2166, y=2) -> (x/y=w2164:dbl[][])
        n718 = Divide(x=w2180, y=2) -> (x/y=w2125:dbl[][])
        n719 = Divide(x=w2173, y=2) -> (x/y=w2127:dbl[][])
        n720 = To Single Precision Float(number=w2160) -> (single precision float=w2159:sgl[][])
        n721 = Transpose 2D Array(2D array=w2164) -> (transposed array=→"Data map":dbl[][])
        n722 = To Single Precision Float(number=w2096) -> (single precision float=w2100:sgl[][])
        n723 = To Single Precision Float(number=w2125) -> (single precision float=w2131:sgl[][])
        n724 = To Single Precision Float(number=w2127) -> (single precision float=w2128:sgl[][])
        n725 = call "IMAQ ArrayToImage"("Image Pixels (Float)"=w2159, "Image"=w2093) -> ("Image Out"=w2162:T2)  [unwired: 8 in, 1 out]
        n726 = call "IMAQ ArrayToImage"("Image Pixels (Float)"=w2100, "Image"=w2092) -> ("Image Out"=w2102:T2)  [unwired: 8 in, 1 out]
        n727 = call "IMAQ ArrayToImage"("Image Pixels (Float)"=w2131, "Image"=w2091) -> ("Image Out"=w2133:T2)  [unwired: 8 in, 1 out]
        n728 = call "IMAQ ArrayToImage"("Image Pixels (Float)"=w2128, "Image"=w2090) -> ("Image Out"=w2130:T2)  [unwired: 8 in, 1 out]
        n729 = call "IMAQ Symmetry"("Type of Symmetry"=w2161, "Image Src"=w2162) -> ("Image Dst Out"=w2157:T2)  [unwired: 3 in, 1 out]
        n730 = call "IMAQ Symmetry"("Type of Symmetry"=w2101, "Image Src"=w2102) -> ("Image Dst Out"=w2098:T2)  [unwired: 3 in, 1 out]
        n731 = call "IMAQ Symmetry"("Type of Symmetry"=w2132, "Image Src"=w2133) -> ("Image Dst Out"=→"Detection Laser X":T2)  [unwired: 3 in, 1 out]
        n732 = call "IMAQ Symmetry"("Type of Symmetry"=w2129, "Image Src"=w2130) -> ("Image Dst Out"=→"Detection Laser Y":T2)  [unwired: 3 in, 1 out]
        n733 = call "IMAQ Set Simple Calibration"("Calibration Axis Info"=T33 {"Origin Pixel"={"X"=0.0, "Y"=0.0}, "Angle Relative to Horizontal (deg)"=0.0, "Axis Reference"=0}, "Grid Descriptor"=T34 {"X Step"=0.3, "Y Step"=0.3, "Unit"=enum."Undefined"}, "Image"=w2157) -> ("Calibrated Image"=→"APD 1":T2)  [unwired: 7 in, 1 out]
        n734 = call "IMAQ Set Simple Calibration"("Calibration Axis Info"=T33 {"Origin Pixel"={"X"=0.0, "Y"=0.0}, "Angle Relative to Horizontal (deg)"=0.0, "Axis Reference"=0}, "Grid Descriptor"=T34 {"X Step"=0.3, "Y Step"=0.3, "Unit"=enum."Undefined"}, "Image"=w2098) -> ("Calibrated Image"=→"APD 2":T2)  [unwired: 7 in, 1 out]
      }
    }
    n735 = Subtract(x=w1064, y="APD 2 Offset") -> (x-y=w1061:waveform(dbl))
    n736 = Subtract(x=w1066, y="APD 1 Offset") -> (x-y=w1062:waveform(dbl))
    n737 = Index Array(array=w1081, index=3) -> (element=w1150:waveform(dbl))
    n738 = Index Array(array=w1081, index=6) -> (element=w1147:waveform(dbl))
    n739 = Build Array(w1062, w1061) -> (→"APD Chart":waveform(dbl)[])
    n740 = Array Size(array=w1139) -> (size(s)=w1194:i32)
    n741 = call <vilib>:"Std Deviation and Variance.vi"("X"=w1074) -> ("standard deviation"=w1073:dbl)  [unwired: 1 in, 2 out]
    n742 = Add Array Elements(numeric array=w1074) -> (sum=w1076:u32)
    n743 = Add Array Elements(numeric array=w1139) -> (sum=w1204:u32)
    n744 = call <vilib>:"Std Deviation and Variance.vi"("X"=w1139) -> ("standard deviation"=w1138:dbl)  [unwired: 1 in, 2 out]
    n745 = Divide(x="T1 offset_x (mV)", y=1000.0) -> (x/y=w1151:dbl)
    n746 = Divide(x=w1073, y=w1072) -> (x/y=w1069:dbl)
    "Rate sigma (Hz) 2" <- w1069
    n747 = Multiply(x=w1072, y=w1194) -> (x*y=w1075:dbl)
    "Int. Time (s)" <- w1075
    n748 = Divide(x=w1076, y=w1075) -> (x/y=w1070:dbl)
    "APD 2 Rate (Hz)" <- w1070
    n749 = Divide(x=w1204, y=w1075) -> (x/y=w1136:dbl)
    "APD 1 Rate (Hz)" <- w1136
    n750 = Divide(x=w1138, y=w1072) -> (x/y=w1137:dbl)
    "Rate sigma (Hz)" <- w1137
    n751 = Divide(x=w1069, y=w1070) -> (x/y=→"Sigma/Mean 2":dbl)
    n752 = Divide(x=w1137, y=w1136) -> (x/y=→"Sigma/Mean":dbl)
    n753 = Divide(x="T2 offset_x (mV)", y=1000.0) -> (x/y=w1149:dbl)
    n754 = case shown="0, Default" "Calibration" {
      tunnel: "T1 alpha_x (nm/V)" -> [_ w2056 w2077]
      tunnel: "T1 kappa_x (pN/nm)" -> [_ _ w2067]
      tunnel: "T2 alpha_x (nm/V)" -> [_ w2055 w2075]
      tunnel: "T2 kappa_x (pN/nm)" -> [_ _ w2068]
      tunnel: w1150 -> [w2038 w2053 w2073]
      tunnel: w1147 -> [w2037 w2051 w2071]
      tunnel: [w2038 w2050 w2070] -> w1180
      tunnel: [w2037 w2049 w2069] -> w1179
      tunnel: ["T1 X (V)" ("Label.Text") "T1 X (nm)" ("Label.Text") "T1 X (pN)" ("Label.Text")] -> w1168
      tunnel: ["T2 X (V)" ("Label.Text") "T2 X (nm)" ("Label.Text") "T2 X (pN)" ("Label.Text")] -> w1167
      tunnel: ["Position (V)" ("Label.Text") "Position (nm)" ("Label.Text") "Force (pN)" ("Label.Text")] -> w1169
      tunnel: w1149 -> [_ w2041 w2060]
      tunnel: w1151 -> [_ w2044 w2062]
      tunnel: ["Mean (V)" ("Label.Text") "Mean (nm)" ("Label.Text") "Mean (pN)" ("Label.Text")] -> w1164
      tunnel: ["Difference (V)" ("Label.Text") "Difference (nm)" ("Label.Text") "Difference (pN)" ("Label.Text")] -> w1089
      frame 0, Default {
      }
      frame 1 {
        # "position"
        n755 = Unbundle By Name(w2053) -> ("Y"=w2057:dbl[])
        n756 = Unbundle By Name(w2051) -> ("Y"=w2042:dbl[])
        n757 = Subtract(x=w2057, y=w2044) -> (x-y=w2045:dbl[])
        n758 = Subtract(x=w2042, y=w2041) -> (x-y=w2043:dbl[])
        n759 = Multiply(x=w2043, y=w2055) -> (x*y=w2052:dbl[])
        n760 = Multiply(x=w2056, y=w2045) -> (x*y=w2054:dbl[])
        n761 = Bundle By Name(cluster=w2051, "Y"=w2052) -> (w2049:waveform(dbl))
        n762 = Bundle By Name(cluster=w2053, "Y"=w2054) -> (w2050:waveform(dbl))
      }
      frame 2 {
        # "force"
        n763 = Unbundle By Name(w2073) -> ("Y"=w2078:dbl[])
        n764 = Unbundle By Name(w2071) -> ("Y"=w2076:dbl[])
        n765 = Subtract(x=w2076, y=w2060) -> (x-y=w2061:dbl[])
        n766 = Subtract(x=w2078, y=w2062) -> (x-y=w2063:dbl[])
        n767 = Compound Arithmetic op=MULTIPLY(w2061, w2075, w2068) -> (w2072:dbl[])
        n768 = Compound Arithmetic op=MULTIPLY(w2067, w2077, w2063) -> (w2074:dbl[])
        n769 = Bundle By Name(cluster=w2071, "Y"=w2072) -> (w2069:waveform(dbl))
        n770 = Bundle By Name(cluster=w2073, "Y"=w2074) -> (w2070:waveform(dbl))
      }
    }
    n771 = feedback-in #17("Calibration") -> ()
    n772 = feedback #17(u16 1 ("Calibration")) -> (w1171:u16)
    n773 = Not Equal?(x=w1171, y="Calibration") -> (x != y?=w1127:bool)
    n774 = Unbundle By Name(w1150) -> ("Y"=w1153:dbl[])
    n775 = Unbundle By Name(w1147) -> ("Y"=w1156:dbl[])
    n776 = Subtract(x=w1153, y=w1151) -> (x-y=w1154:dbl[])
    n777 = Subtract(x=w1156, y=w1149) -> (x-y=w1155:dbl[])
    n778 = Multiply(x=w1155, y="T2 alpha_x (nm/V)") -> (x*y=w1146:dbl[])
    n779 = Multiply(x="T1 alpha_x (nm/V)", y=w1154) -> (x*y=w1145:dbl[])
    n780 = Multiply(x=w1179, y=-1.0) -> (x*y=w1158:waveform(dbl))
    n781 = case shown="True" "Read Lateness and Rel Phase" {
      tunnel: w981 -> [w1613 w1635]
      tunnel: w980 -> [w1614 w1634]
      tunnel: [w1613 w1633] -> w1142
      tunnel: [w1614 w1632] -> w1141
      frame False {
      }
      frame True {
        n782 = xnode "Read/Write Control"("FPGA VI Reference In"=w1635, "error in"=w1634) -> ("FPGA VI Reference Out"=w1633:T19, "error out"=w1632:errorcluster, "GI Relative phase"=→"GI relative phase":i16, "Relative phase"=→"Relative phase (AI1)":i16, "AI Late Counter"=→"Late Counter (AI1)":u16, "GI Late Counter"=→"GI Late Counter":u16, "MCL Late Counter"=→"MCL Late Counter":u16, "MCL Relative Phase"=→"Relative Phase (MCL)":i16, "APD Acq Relative Phase"=→"APD Acq Relative Phase":i16, "APD 1 Gate Relative Phase"=→"APD 1 Gate Relative Phase":i16, "APD 2 Gate Relative Phase"=→"APD 2 Gate Relative Phase":i16, "APD Acq Late Counter"=→"APD Acq Late Counter":u16, "APD 1 Gate Late Counter"=→"APD 1 Gate Late Counter":u16, "APD 2 Gate Late Counter"=→"APD 2 Gate Late Counter":u16, "Green FB Relative Phase"=→"Relative phase (Green FB)":i16, "GI Relative phase 2"=→"GI relative phase 2":i16, "GI Late Counter 2"=→"GI Late Counter 2":u16, "Trap Pos FIFO Timeout"=→"Trap Pos FIFO Timeout":u16, "Trap AI FIFO Timeout"=→"Trap AI FIFO Timeout":u16)
      }
    }
    n783 = Subtract(x=w1146, y=w1145) -> (x-y=w1144:dbl[])
    n784 = Unbundle By Name(w1179) -> ("Y"=w1114:dbl[])
    n785 = Unbundle By Name(w1180) -> ("Y"=w1115:dbl[])
    n786 = Build Array(w1180, w1158) -> (→"Force":waveform(dbl)[])
    n787 = Subtract(x=w1144, y="Offset (nm)") -> (x-y=w1112:dbl[])
    n788 = call <vilib>:"Mean.vi"("X"=w1114) -> ("mean"=w1093:dbl)  [unwired: 1 out]